vi "PowerSpectrum.vi"(10 "Array":dbl[][](array[numeric])=array100000x5[500000 elements]) -> ()   [LabVIEW 2010]
uses:
  <vilib>/Analysis/2dsp.llb/Power Spectrum (DBL).vi
  <vilib>/Analysis/NI_AALPro.lvlib
  <vilib>/Analysis/NI_AALBase.lvlib
panel:
  in  "Save Data and Close":bool
  in  "stop":bool
  in  "Save Spectrum":bool
  in  "Show:":u16(ring) items=["Particle 1"]
  out "stiffness/N/m":dbl[](array[numeric])=[1.1635155358729046e-05, 1.0687249343003817e-05] format="%#_3p"
  out "standard deviation/m":dbl[](array[numeric])=[1.8863143875454795e-08, 1.9681908096730664e-08] format="%#_3p"
  in  "# bins":u32=100
  in  "minimum frequency/Hz":dbl=1.0
  out "camera speed/Hz":dbl=3880.0294882239527 format="%#.0f"
  out "Scatterplot":cluster{dbl[], dbl[]}(graph)
  out "Power Spectrum":cluster{dbl[], dbl[]}[](graph)=[{[1.0282078143793476, 1.1058084041438265, 1.2028091413494255, 1.2998098785550243, 1.396810615760623, 1.5132115004073416, 1.6296123850540603, 1.7654134171418987, 1.901214449229737, 2.0370154813175754, 2.211616808287653, 2.386218135257731, 2.560819462227809, 2.7742210840801262, 3.0070228533735635, 3.2398246226670007, 3.4920265394015577, 3.7636286035772346, 4.054630815194031, 4.384433321693067, 4.733635975633223, 5.102238777014498, 5.509641873278014, 5.936445116982648, 6.402048655569523, 6.906452489038636, 7.44965661738999, 8.031661040623582, 8.652465758739416, 9.331470919178606, 10.068676521941159, 10.864082567027069, 11.717689054436338, 12.648896131610087, 13.638303651107195, 14.705311760368781, 15.869320606835968, 17.110930043067633, 18.449540216504897, 19.90455127458888, 21.47596321731958, 23.163776044697, 24.987389904162256, 26.946804795715355, 29.06142086679741, 31.35063826484954, 33.81445698987175, 36.47227718930516, 39.34349901059088, 42.44752260117004, 45.78434796104265, 49.3733752376498, 53.25340472587376, 57.44383657315562, 61.96407092693653, 66.83350793465759, 72.09094789120105, 77.77519109144914, 83.88623753540186, 90.48228766538259, 97.60214177627354, 105.26520001551584, 113.54906297287398, 122.4925309432302, 132.1150040740256, 142.49408295502468, 153.7073681759919, 165.7936600318095, 178.83055911224199, 192.89566600705382, 208.06658130600948, 224.44030574631455, 242.09443991773355, 261.12598455747207, 281.65134055017677, 303.8063089279355, 327.70729057539506, 353.4706863772021, 381.27109766032675, 411.2637256042979, 443.60377138864453, 478.4852364877779, 516.1215225235502, 556.7066309703728, 600.473363597539, 647.7127226166656, 698.6575097970461, 753.5987273502973, 812.8661777829182, 876.7896636014078, 945.7377876071474, 1020.1179528964007, 1100.356962712872, 1186.8816203002661, 1280.2157296394932, 1380.902494858905, 1489.5045202342933, 1606.6426104837744, 1732.9957707677875, 1869.2818065416539], [15.072001545838193, 5.381064208181686, 20.802723375926206, 12.102989660424853, 12.391970853921608, 10.934968512925145, 13.20903342733509, 9.12318125085424, 6.533629236464283, 5.728531488354745, 7.13169334867029, 7.4993769990386925, 6.293750354616378, 12.703692788970432, 4.47899718296089, 13.27470181232107, 7.5232172267102975, 4.0381288096011, 10.23307253567812, 3.1548237707603737, 8.277396753882668, 9.018893523545406, 5.112218185000436, 4.157128607816847, 5.70076799857964, 4.123623421741239, 5.350370546150154, 3.683496581050495, 4.008526840792756, 5.676198081744598, 3.8470614845135507, 4.976043687160064, 3.6062742929219054, 2.8013853348409006, 2.947101032957517, 2.9881877435636195, 2.7630441641741785, 3.9411981399866716, 2.40538554055038, 2.912461194160887, 2.9891982063983233, 2.985136416248091, 1.9406573670686258, 2.3731411757133385, 2.267565832737222, 1.9966843359447848, 2.282461555549319, 1.867761086026223, 1.7029422727863701, 1.5980378733963518, 1.3769976566454014, 1.6395976744645695, 1.3713666590664095, 1.318128425757895, 1.3646956445470948, 1.2695829213560192, 1.0468559580863739, 0.9777364341541396, 0.9919431125185824, 0.8961836407662447, 0.7798830824213393, 0.7754331416955393, 3.3319414426740974, 0.5908270275541873, 0.5205353031330278, 0.4071109350227232, 0.34257776570487125, 0.35694825490300686, 0.28550212278673276, 0.26858533981735166, 0.23270831150923862, 0.22857191892780718, 0.1772015429392824, 0.17235607020464971, 0.13531606966154425, 0.10795798302327796, 0.10346960883763362, 0.20470546349109092, 0.0758351105518506, 0.061241119050297804, 0.05444489066318583, 0.051072628083504816, 0.04291472820006293, 0.034910575243884065, 0.03079833924755271, 0.02798861372197582, 0.02331486724852399, 0.020827582304554455, 0.017288398787854174, 0.015788024624458587, 0.01434570739503853, 0.012807584790698882, 0.010829004781237096, 0.009985417882284362, 0.009176817140394556, 0.008256479791359178, 0.008040360384750101, 0.006909623918801784, 0.006571388135605079, 0.006326119377659595]}, {[1.0282078143793476, 1.1058084041438265, 1.2028091413494255, 1.2998098785550243, 1.396810615760623, 1.5132115004073416, 1.6296123850540603, 1.7654134171418987, 1.901214449229737, 2.0370154813175754, 2.211616808287653, 2.386218135257731, 2.560819462227809, 2.7742210840801262, 3.0070228533735635, 3.2398246226670007, 3.4920265394015577, 3.7636286035772346, 4.054630815194031, 4.384433321693067, 4.733635975633223, 5.102238777014498, 5.509641873278014, 5.936445116982648, 6.402048655569523, 6.906452489038636, 7.44965661738999, 8.031661040623582, 8.652465758739416, 9.331470919178606, 10.068676521941159, 10.864082567027069, 11.717689054436338, 12.648896131610087, 13.638303651107195, 14.705311760368781, 15.869320606835968, 17.110930043067633, 18.449540216504897, 19.90455127458888, 21.47596321731958, 23.163776044697, 24.987389904162256, 26.946804795715355, 29.06142086679741, 31.35063826484954, 33.81445698987175, 36.47227718930516, 39.34349901059088, 42.44752260117004, 45.78434796104265, 49.3733752376498, 53.25340472587376, 57.44383657315562, 61.96407092693653, 66.83350793465759, 72.09094789120105, 77.77519109144914, 83.88623753540186, 90.48228766538259, 97.60214177627354, 105.26520001551584, 113.54906297287398, 122.4925309432302, 132.1150040740256, 142.49408295502468, 153.7073681759919, 165.7936600318095, 178.83055911224199, 192.89566600705382, 208.06658130600948, 224.44030574631455, 242.09443991773355, 261.12598455747207, 281.65134055017677, 303.8063089279355, 327.70729057539506, 353.4706863772021, 381.27109766032675, 411.2637256042979, 443.60377138864453, 478.4852364877779, 516.1215225235502, 556.7066309703728, 600.473363597539, 647.7127226166656, 698.6575097970461, 753.5987273502973, 812.8661777829182, 876.7896636014078, 945.7377876071474, 1020.1179528964007, 1100.356962712872, 1186.8816203002661, 1280.2157296394932, 1380.902494858905, 1489.5045202342933, 1606.6426104837744, 1732.9957707677875, 1869.2818065416539], [11.25935335990701, 14.974595661648634, 6.998339566491533, 14.085523115503712, 14.553303410772907, 19.097323989309956, 17.006038691614673, 19.23863625219445, 4.543729694036814, 8.554321584183146, 11.046198817892755, 4.539061006488037, 3.174332827077048, 7.917588724092648, 8.362419314554609, 7.0362029654588945, 4.8818943404900175, 7.745710652033042, 6.028156046530081, 6.876043836724806, 14.219513400049108, 9.909210902274554, 6.099494158153199, 7.79968188909321, 7.9389914834929405, 3.6567125896739783, 3.162465529661849, 7.057854390344928, 6.269286281133227, 4.608778749059326, 5.300596444820996, 6.158249903118502, 4.3039574888668515, 3.757395541890763, 2.908255103356603, 4.759750903839909, 4.313175512981051, 3.7131611021618345, 3.78392201328176, 4.839700262323097, 2.916641846189601, 2.4353614444880085, 2.4723095955150347, 3.1483932052079497, 2.9913885067478327, 2.6029377619314418, 3.0737412779266156, 2.3084512663249894, 2.289553688478108, 2.1836073902902933, 1.8414138904867574, 2.04779107991743, 1.5989018567830384, 1.4189322465506748, 1.518350949815974, 1.44517607213078, 1.3579727190658513, 1.0700768728532384, 1.1960451453364083, 1.0488620722213706, 0.9051890023155346, 0.8456992892615144, 1.576628598132485, 0.655959936304109, 0.5330941292551482, 0.4991899991862849, 0.4236812548410148, 0.3779582084314599, 0.2963960527320926, 0.2808182000626122, 0.24476860680360527, 0.30042173591219606, 0.19889215042272299, 0.16888376489275875, 0.14538684099575594, 0.11864487913047626, 0.10139206755498278, 0.09324504020437822, 0.0800792595581277, 0.0638898756847623, 0.05955565320509185, 0.05359466329803577, 0.04740343943737344, 0.03901789789034158, 0.033873824585791815, 0.031743919697078786, 0.023583436487443783, 0.02200443505431703, 0.020085239904671932, 0.017845091367584488, 0.014604835833478831, 0.013248862230663693, 0.012967988650149215, 0.01079339725610198, 0.009344834332284814, 0.008884105079382434, 0.009275241721965873, 0.008456925460095657, 0.008385676077730405, 0.006840897376814484]}]
  # "N.B. The format for data files is tab delimited, one frame per line, with columns which are: time/s, then x/um, y/um for each particle"
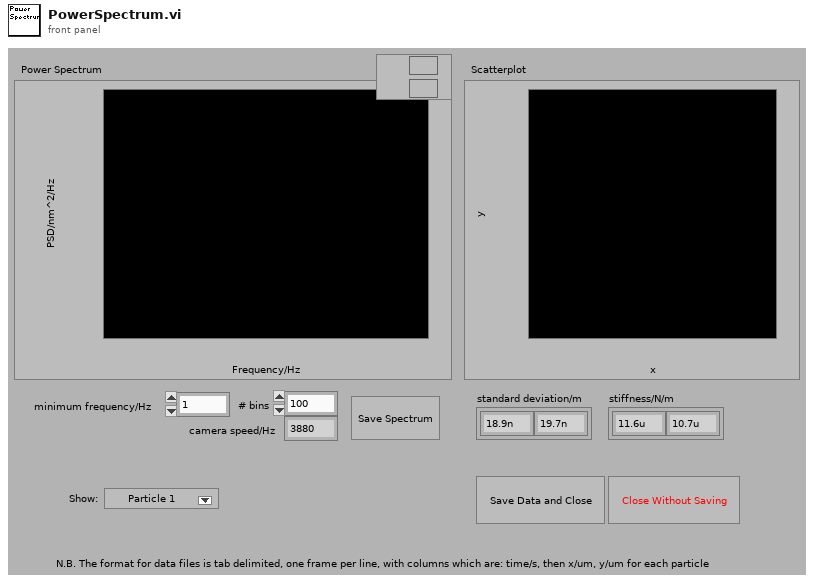
[diagram p1: front panel]
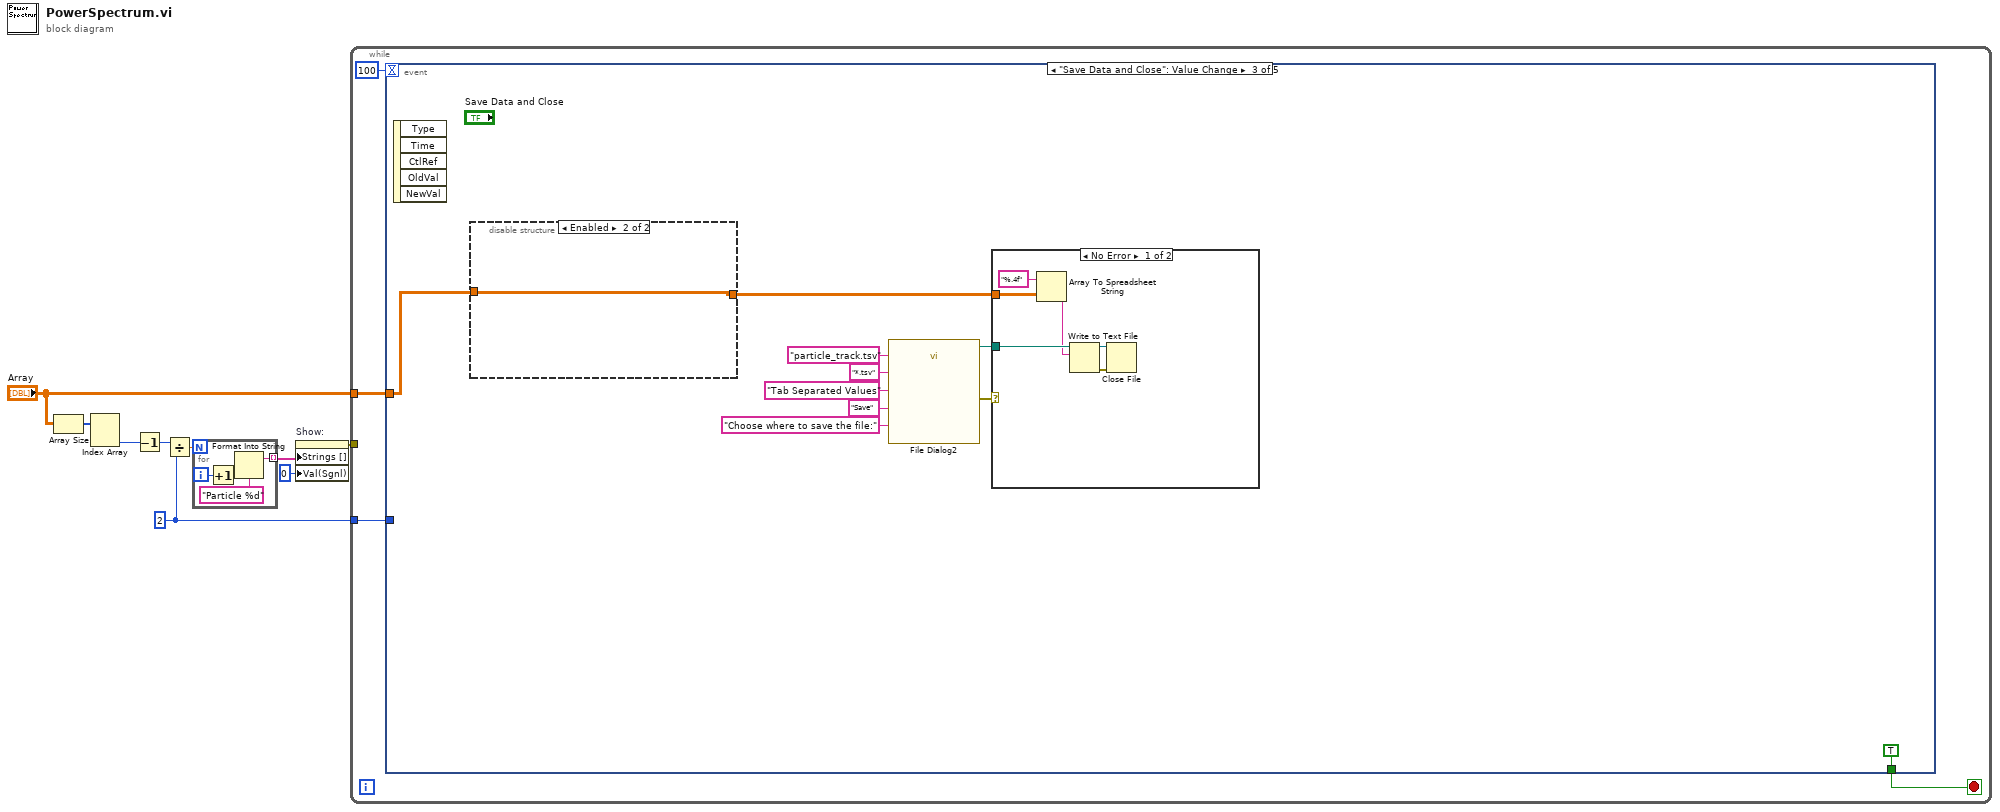
[diagram p0: block diagram]
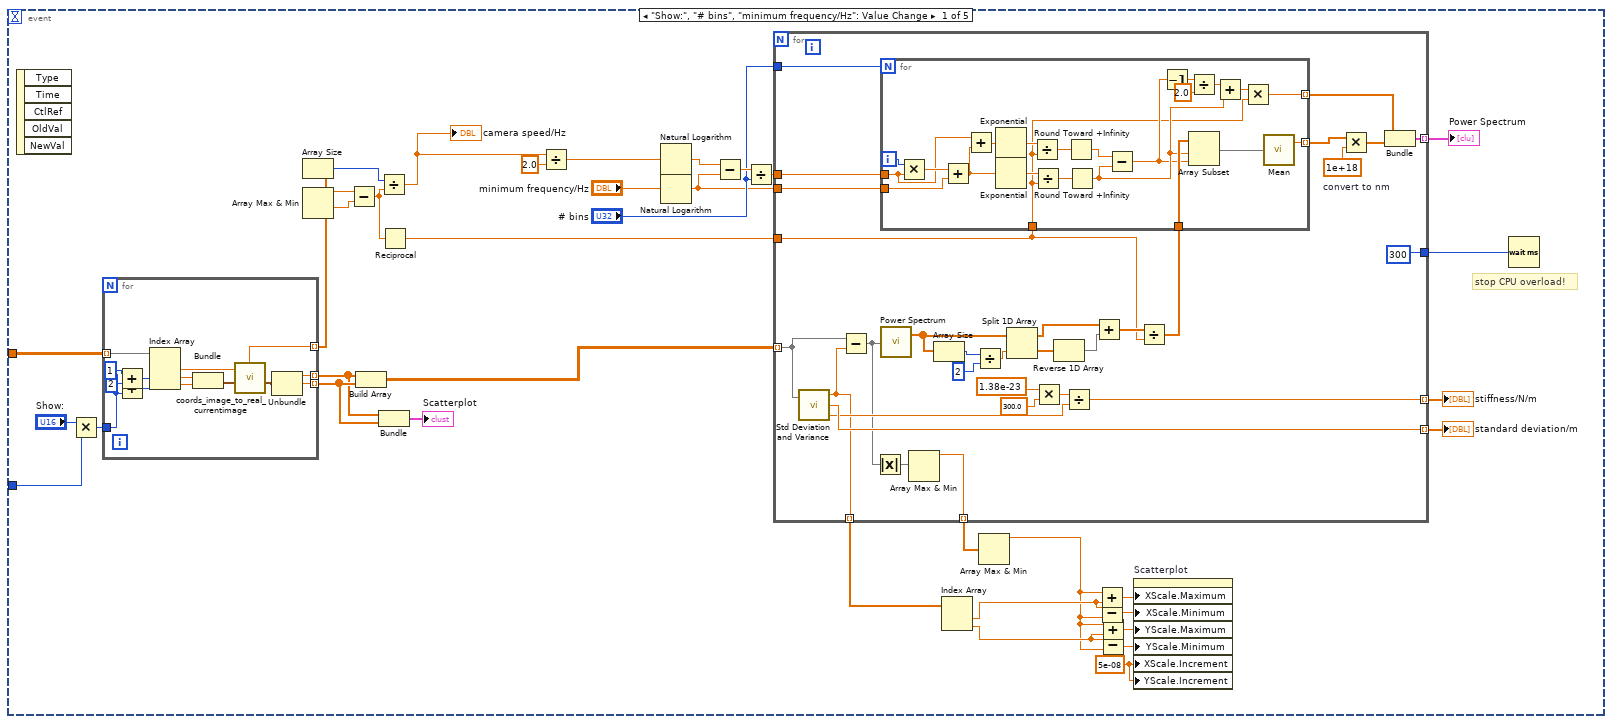
[diagram p2: hidden frame]
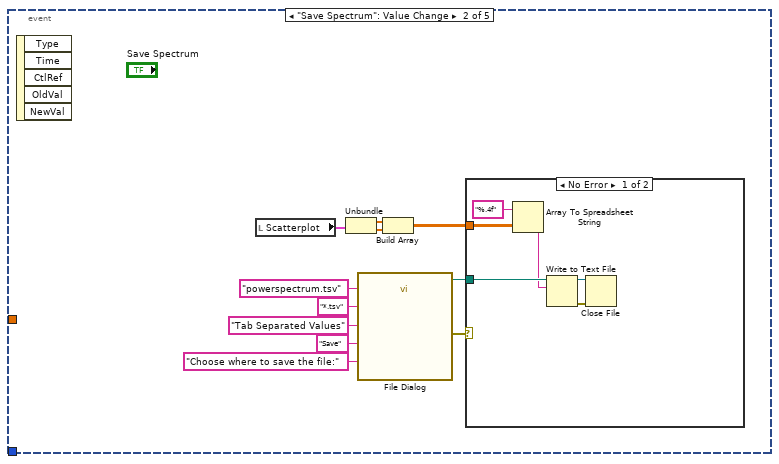
[diagram p3: hidden frame]
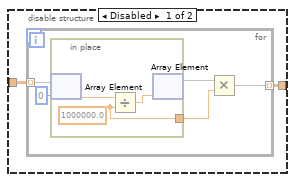
[diagram p5: hidden frame]
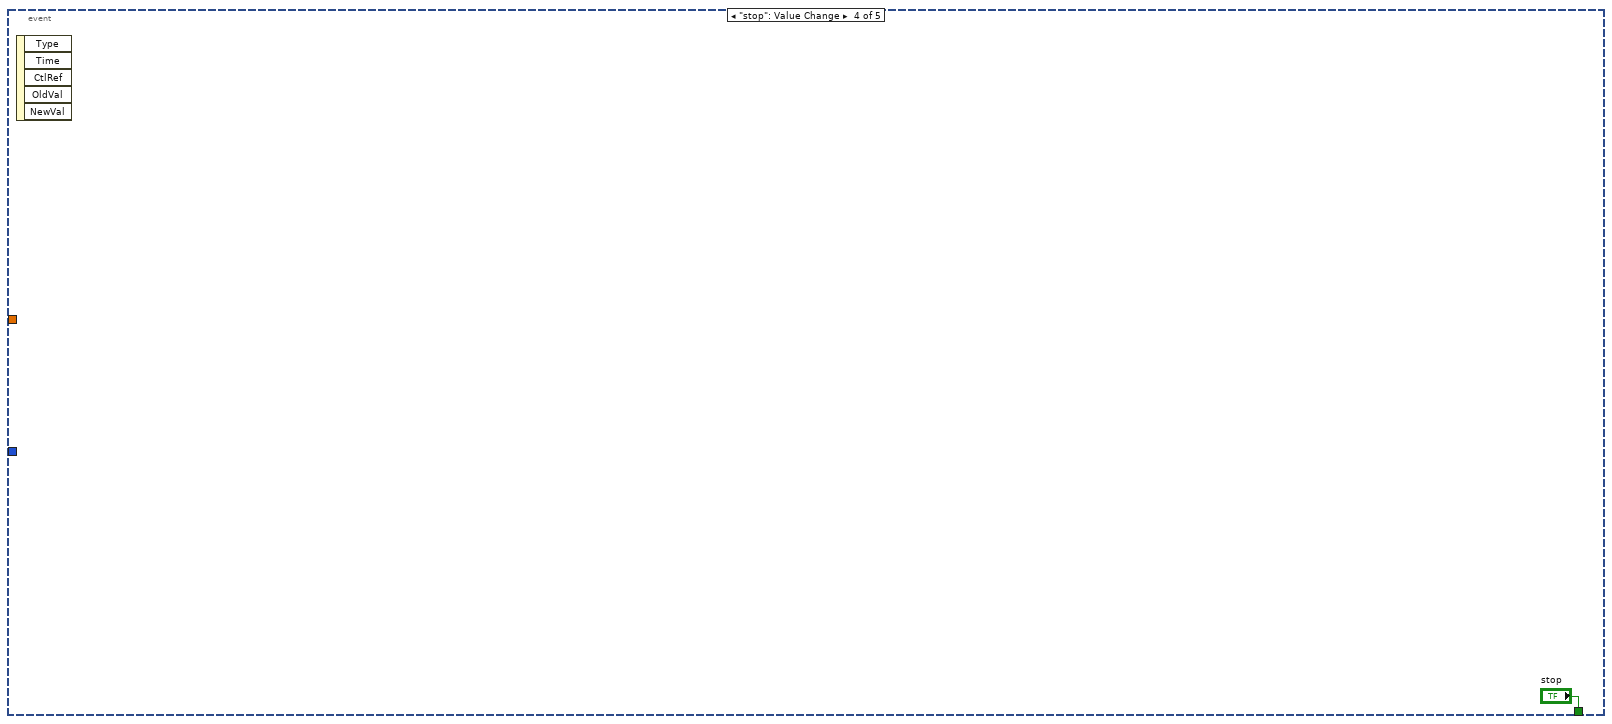
[diagram p7: hidden frame]
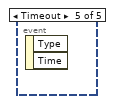
[diagram p8: hidden frame]
diagram:
  w2 = 2 ("y")
  n1 = Array Size(array="Array") -> (size(s)=w8:i32[])
  n2 = Index Array(array=w8) -> (element #2=w7:i32)  [unwired: 2 in, 1 out]
  n3 = Decrement(x=w7) -> (x-1=w5:i32)
  n4 = Divide(x=w5, y=w2) -> (x/y=w4:dbl)
  n5 = for {
    N: w4 -> [_]
    tunnel: [w11] -> w6 mode=indexing
    i -> [w13]
    n6 = Increment(x=w13) -> (x+1=w10:i32)
    n7 = Format Into String(format string="Particle %d", w10) -> (resulting string=w11:string)  [unwired: 2 in, 1 out]
  }
  n8 = property on="Show:" class="Ring (strict)"("Strings []"=w6, "Val(Sgnl)"=u16 0 ("Value (Signaling)")) -> (error out=w3:errorcluster)  [unwired: 2 in, 1 out]
  n9 = while {
    tunnel: "Array" -> [w17]
    tunnel: w3 -> [_]
    tunnel: w2 -> [w16]
    stop <- w14 stop-if-true
    n10 = event shown="[2] \"Save Data and Close\": Value Change" {
      selector: _ -> [_ _ _ _ _]
      dyn-events: _ -> [_ _ _ _ _]
      timeout: 100 -> [_ _ _ _ _]
      tunnel: w17 -> [w22 _ w139 _ _]
      tunnel: w16 -> [w21 _ _ _ _]
      tunnel: [_ _ TRUE ("stop") "stop" _] -> w14
      event "Show:", "# bins", "minimum frequency/Hz": Value Change {
        w23 = 5e-08 ("X Scale.Range:Increment")
        # "stop CPU overload!"
        n11 = event-data() -> ()  [unwired: 1 in, 5 out]
        n12 = Multiply(x="Show:", y=w21) -> (x*y=w20:i32)
        n13 = for {
          tunnel: w22 -> [w119] mode=indexing
          tunnel: [w114] -> w34 mode=indexing
          tunnel: [w113] -> w39 mode=indexing
          tunnel: [w112] -> w51 mode=indexing
          tunnel: w20 -> [w109]
          n14 = Add(x=1, y=w109) -> (x+y=w111:i32)
          n15 = Add(x=2, y=w109) -> (x+y=w110:i32)
          n16 = Index Array(array=w119, index #2=w111, index #3=w110) -> (element #1=w112:dbl, element #2=w118:dbl, element #3=w117:dbl)  [unwired: 1 in]
          n17 = Bundle(w118, w117) -> (w116:cluster{dbl, dbl})  [unwired: 1 in]
          n18 = call "coords_image_to_real_currentimage.vi"("Position (pixels on image)"=w116) -> ("Position (real coords)"=w115:cluster{dbl, dbl, "Z":dbl})  [unwired: 9 in]
          n19 = Unbundle(w115) -> (w114:dbl, w113:dbl)  [unwired: 1 out]
        }
        n20 = Array Size(array=w51) -> (size(s)=w50:i32)
        n21 = Array Max & Min(array=w51) -> (max value=w53:dbl, min value=w52:dbl)  [unwired: 2 out]
        n22 = Subtract(x=w53, y=w52) -> (x-y=w49:dbl)
        n23 = Build Array(w34, w39) -> (w38:dbl[][])
        n24 = Divide(x=w50, y=w49) -> (x/y=w33:dbl)
        "camera speed/Hz" <- w33
        n25 = Bundle(w34, w39) -> (→"Scatterplot":cluster{dbl[], dbl[]})  [unwired: 1 in]
        n26 = Reciprocal(x=w49) -> (1/x=w41:dbl)
        n27 = Divide(x=w33, y=2.0) -> (x/y=w35:dbl)
        n28 = Natural Logarithm(1:w35) -> (0:w46:dbl)
        n29 = Natural Logarithm(1:"minimum frequency/Hz") -> (0:w42:dbl)
        n30 = Subtract(x=w46, y=w42) -> (x-y=w45:dbl)
        n31 = Divide(x=w45, y="# bins") -> (x/y=w43:dbl)
        n32 = for {
          tunnel: "# bins" -> [w77]
          tunnel: w43 -> [w76]
          tunnel: w42 -> [w75]
          tunnel: w41 -> [w61]
          tunnel: [w71] -> w37 mode=indexing
          tunnel: [w70] -> w36 mode=indexing
          tunnel: [w69] -> w40 mode=indexing
          tunnel: w38 -> [w59] mode=indexing
          tunnel: [w60] -> w31 mode=indexing
          tunnel: [w56] -> w32 mode=indexing
          tunnel: [u32 300 ("milliseconds to wait")] -> w18
          w66 = 1e+18  # convert to nm
          n33 = call <vilib>:"Std Deviation and Variance.vi"("X"=w59) -> ("mean"=w60:dbl, "standard deviation"=w71:dbl, "variance"=w64:dbl)  [unwired: 1 in]
          n34 = Subtract(x=w59, y=w60) -> (x-y=w57:dbl[])
          n35 = Absolute Value(x=w57) -> (abs(x)=w58:dbl[])
          n36 = call-poly <vilib>:"Power Spectrum.vi"("X"=w57) -> ("Power Spectrum"=w84:dbl[])  [unwired: 1 out]
          n37 = Array Max & Min(array=w58) -> (max value=w56:dbl)  [unwired: 3 out]
          n38 = Array Size(array=w84) -> (size(s)=w83:i32)
          n39 = Divide(x=w83, y=2) -> (x/y=w78:dbl)
          n40 = Split 1D Array(array=w84, index=w78) -> (first subarray=w80:dbl[], second subarray=w81:dbl[])
          n41 = Multiply(x=1.38e-23 ("1/x"), y=300.0 ("1/x")) -> (x*y=w72:dbl)
          n42 = Reverse 1D Array(array=w81) -> (reversed array=w79:dbl[])
          n43 = Divide(x=w72, y=w64) -> (x/y=w70:dbl)
          n44 = Add(x=w80, y=w79) -> (x+y=w62:dbl[])
          n45 = Divide(x=w62, y=w61) -> (x/y=w63:dbl[])
          n46 = for {
            N: w77 -> [_]
            tunnel: w76 -> [w100]
            tunnel: w75 -> [w104]
            tunnel: w61 -> [w85]
            tunnel: w63 -> [w95]
            tunnel: [w89] -> w67 mode=indexing
            tunnel: [w87] -> w68 mode=indexing
            i -> [w106]
            n47 = Multiply(x=w106, y=w100) -> (x*y=w105:dbl)
            n48 = Add(x=w105, y=w104) -> (x+y=w101:dbl)
            n49 = Add(x=w100, y=w101) -> (x+y=w99:dbl)
            n50 = Exponential(1:w99) -> (0:w98:dbl)
            n51 = Exponential(1:w101) -> (0:w103:dbl)
            n52 = Divide(x=w98, y=w85) -> (x/y=w97:dbl)
            n53 = Divide(x=w103, y=w85) -> (x/y=w102:dbl)
            n54 = Round Toward +Infinity(x=w97) -> (ceil(x): smallest int >= x=w96:dbl)
            n55 = Round Toward +Infinity(x=w102) -> (ceil(x): smallest int >= x=w91:dbl)
            n56 = Subtract(x=w96, y=w91) -> (x-y=w86:dbl)
            n57 = Decrement(x=w86) -> (x-1=w94:dbl)
            n58 = Divide(x=w94, y=2.0) -> (x/y=w92:dbl)
            n59 = Array Subset(array=w95, index=w91, length=w86) -> (w88:dbl[])
            n60 = Add(x=w92, y=w91) -> (x+y=w90:dbl)
            n61 = Multiply(x=w90, y=w85) -> (x*y=w89:dbl)
            n62 = call <vilib>:"Mean.vi"("X"=w88) -> ("mean"=w87:dbl)  [unwired: 1 out]
          }
          n63 = Multiply(x=w68, y=w66) -> (x*y=w65:dbl[])
          n64 = Bundle(w67, w65) -> (w69:cluster{dbl[], dbl[]})  [unwired: 1 in]
        }
        "Power Spectrum" <- w40
        "standard deviation/m" <- w37
        "stiffness/N/m" <- w36
        n65 = Index Array(array=w31) -> (element #1=w25:dbl, element #2=w26:dbl)  [unwired: 2 in]
        n66 = Array Max & Min(array=w32) -> (max value=w24:dbl)  [unwired: 3 out]
        n67 = Add(x=w24, y=w25) -> (x+y=w29:dbl)
        n68 = Subtract(x=w25, y=w24) -> (x-y=w30:dbl)
        n69 = Add(x=w24, y=w26) -> (x+y=w28:dbl)
        n70 = Subtract(x=w26, y=w24) -> (x-y=w27:dbl)
        n71 = property on="Scatterplot" class="XYGraph (strict)"("XScale.Maximum"=w29, "XScale.Minimum"=w30, "YScale.Maximum"=w28, "YScale.Minimum"=w27, "XScale.Increment"=w23, "YScale.Increment"=w23) -> ()  [unwired: 2 in, 2 out]
        n72 = Wait (ms)(milliseconds to wait=w18) -> ()  [unwired: 1 out]
      }
      event "Save Spectrum": Value Change {
        n73 = event-data() -> ()  [unwired: 1 in, 5 out]
        n74 = local read "Scatterplot"() -> (w130:cluster{dbl[], dbl[]})
        n75 = Unbundle(w130) -> (w128:dbl[], w129:dbl[])
        n76 = call "File Dialog"("prompt"="Choose where to save the file:", "button label"="Save", "default name"="powerspectrum.tsv", "pattern (all files)"="*.tsv", "pattern label"="Tab Separated Values") -> ("selected path"=w121:path, "error out"=w120:errorcluster)  [unwired: 7 in, 2 out]
        n77 = Build Array(w128, w129) -> (w127:dbl[][])
        n78 = case shown="No Error" w120 {
          tunnel: w127 -> [w136 _]
          tunnel: w121 -> [w132 _]
          frame No Error {
            n79 = Array To Spreadsheet String(array=w136, 3:"%.4f" ("format string")) -> (spreadsheet string=w131:string)  [unwired: 1 in]
            n80 = Write to Text File(file (use dialog)=w132, text=w131) -> (refnum out=w133:refnum<file>, error out=w134:errorcluster)  [unwired: 2 in, 1 out]
            n81 = Close File(refnum=w133, error in=w134) -> ()  [unwired: 2 out]
          }
          frame Error {
          }
        }
      }
      event "Save Data and Close": Value Change {
        n82 = event-data() -> ()  [unwired: 1 in, 5 out]
        n83 = disable-structure shown="Enabled" {
          disable-tunnel: w139 -> [w148 w157]
          disable-tunnel: [w147 w157] -> w138
          frame Disabled {
            n84 = for {
              tunnel: w148 -> [w153] mode=indexing
              tunnel: [w149] -> w147 mode=indexing
              n85 = in-place {
                in-place-border: [w154] -> w150
                w154 = 1000000.0 ("y")
                n86 = in-place-array #1(w153, 0) -> (w156:dbl)
                n87 = Divide(x=w156, y=w154) -> (x/y=w155:dbl)
                n88 = in-place-array #1(w155) -> (w151:dbl[])  [unwired: 1 out]
              }
              n89 = Multiply(x=w151, y=w150) -> (x*y=w149:dbl[])
            }
          }
          frame Enabled {
          }
        }
        n90 = call "File Dialog2"("prompt"="Choose where to save the file:", "button label"="Save", "default name"="particle_track.tsv", "pattern (all files)"="*.tsv", "pattern label"="Tab Separated Values") -> ("selected path"=w141:path, "error out"=w140:errorcluster)  [unwired: 7 in, 2 out]
        n91 = case shown="No Error" w140 {
          tunnel: w138 -> [w163 _]
          tunnel: w141 -> [w159 _]
          frame No Error {
            n92 = Array To Spreadsheet String(array=w163, 3:"%.4f" ("format string")) -> (spreadsheet string=w158:string)  [unwired: 1 in]
            n93 = Write to Text File(file (use dialog)=w159, text=w158) -> (refnum out=w160:refnum<file>, error out=w161:errorcluster)  [unwired: 2 in, 1 out]
            n94 = Close File(refnum=w160, error in=w161) -> ()  [unwired: 2 out]
          }
          frame Error {
          }
        }
      }
      event "stop": Value Change {
        n95 = event-data() -> ()  [unwired: 1 in, 5 out]
      }
      event Timeout {
        n96 = event-data() -> ()  [unwired: 1 in, 2 out]
      }
    }
  }
